vi "SMain.vi"() -> ()   [LabVIEW 2011] (continued)
-2.431327\t-2.435970\t-2.438255\t-2.439214\t-2.441636\t-2.442908\t-2.443591\t-2.444271\t-2.446042\t-2.447553\t-2.451574\t-2.454322\t-2.459259\t-2.459167\t-2.458988\t-2.459791\t-2.459803\t-2.460155\t-2.460693\t-2.460836\t-2.461752\t-2.464313\t-2.467197\t-2.467691\t-2.467576\t-2.466714\t-2.466182\t-2.465541\t-2.466343\t-2.466851\t-2.466728\t-2.468352\t-2.469074\t-2.468673\t-2.470402\t-2.472062\t-2.472489\t-2.471700\t-2.474044\t-2.476117\t-2.475176\t-2.475954\t-2.477194\t-2.478101\t-2.478769\t-2.482395\t-2.482993\t-2.485696\t-2.489882\t-2.491889\t-2.493382\t-2.496300\t-2.497217\t-2.495696\t-2.497921\t-2.498425\t-2.499485\t-2.502473\t-2.505013\t-2.507983\t-2.511344\t-2.514346\t-2.515093\t-2.515869\t-2.515267\t-2.517344\t-2.516297\t-2.517832\t-2.521177\t-2.524304\t-2.525843\t-2.529733\t-2.532366\t-2.533173\t-2.533271\t-2.533655\t-2.534038\t-2.534921\t-2.537768\t-2.538384\t-2.540839\t-2.543183\t-2.545565\t-2.547411\t-2.547801\t-2.550262\t-2.549876\t-2.551255\t-2.551288\t-2.551510\t-2.553730\t-2.556228\t-2.557870\t-2.560246\t-2.561557\t-2.564050\t-2.564885\t-2.566860\t-2.568948\t-2.568611\t-2.571201\t-2.573409\t-2.574788\t-2.577568\t-2.579327\t-2.581748\t-2.583365\t-2.586189\t-2.588238\t-2.588712\t-2.590200\t-2.592187\t-2.593757\t-2.594959\t-2.595729\t-2.597616\t-2.599509\t-2.602154\t-2.604658\t-2.607614\t-2.609660\t-2.610898\t-2.612830\t-2.613601\t-2.613473\t-2.613544\t-2.616515\t-2.620266\t-2.623817\t-2.625905\t-2.631148\t-2.636015\t-2.640186\t-2.641079\t-2.645126\t-2.645173\t-2.647065\t-2.649247\t-2.651238\t-2.654179\t-2.659284\t-2.665190\t-2.667742\t-2.672541\t-2.674807\t-2.673944\t-2.674205\t-2.673847\t-2.674862\t-2.676190\t-2.680985\t-2.685422\t-2.692200\t-2.698753\t-2.698318\t-2.697628\t-2.696863\t-2.697049\t-2.696832\t-2.697279\t-2.698751\t-2.702908\t-2.706973\t-2.710686\t-2.713145\t-2.713343\t-2.712896\t-2.711070\t-2.708909\t-2.707335\t-2.707843\t-2.708280\t-2.711253\t-2.715050\t-2.720516\t-2.723712\t-2.725368\t-2.726278\t-2.724675\t-2.723140\t-2.723831\t-2.722631\t-2.724579\t-2.727613\t-2.731521\t-2.734936\t-2.739656\t-2.743268\t-2.746792\t-2.750426\t-2.752496\t-2.755723\t-2.757728\t-2.759774\t-2.761461\t-2.765547\t-2.772756\t-2.778340\t-2.784959\t-2.791224\t-2.797387\t-2.800765\t-2.804883\t-2.808755\t-2.808718\t-2.813039\t-2.817153\t-2.823224\t-2.831411\t-2.838495\t-2.843969\t-2.849768\t-2.853002\t-2.856091\t-2.857814\t-2.858783\t-2.860619\t-2.865346\t-2.870363\t-2.877086\t-2.881230\t-2.886957\t-2.887244\t-2.886706\t-2.885127\t-2.880446\t-2.879572\t-2.879982\t-2.883966\t-2.885899\t-2.890801\t-2.894663\t-2.892103\t-2.888604\t-2.883640\t-2.878263\t-2.874808\t-2.869963\t-2.868088\t-2.865550\t-2.867525\t-2.869974\t-2.869190\t-2.870537\t-2.869512\t-2.866932\t-2.865189\t-2.861443"]
  in  "Impedance Spec String 2":string="@;@"
  in  "Data Points 2":i32
  in  "Compensation(ohm) 2":dbl
  in  "StopTimeNs 2":dbl
  in  "Start TimeNs 2":dbl
  in  "Impedance Filter 2":bool
  in  "Filter Risetime(ps) 2":dbl min=1.0 max=1000.0 step=1.0
  out "width2":i32
  out "width1":i32
  out "auto get refer point":bool
  out "SystemMode":string="GPF001"
  out "Count":i16=1
  out "DateCode8Value_0X30":i32=32 format="%x"
  out "ConvertStyle":bool
  out "CountXmlPath":path=path "D:/高频房软件/2. HPTS_VNA_Rev2.7.1.3-1107最新源码/DataBase/L99QF015-SD-R/20161114.xml"
  out "PassCount?":bool=TRUE
  out "upload":bool
  out "AlarmDisplay":bool=TRUE
  out "NetPathCompress2":path=path "\\\\172.20.20.113\\emc/HPTS/SI"
  out "NetPathCompress1":path=path "\\\\172.20.20.113\\emc/HPTS/VNA"
  out "NetCmdCompress":string="net use \\\\172.20.20.113 mesuser /user:mesuser"
  out "NetPathHW":string="\\\\172.20.20.86\\HuaweiData\\DataRoot\\XML"
  out "NetCmd":string="net use \\\\172.20.20.86 Luxshare-ict /user:C040345"
  out "NEXTList":string[](array[string])=["TX1-RX1", "TX2-RX1", "TX3-RX1", "TX4-RX1", "TX1-RX2", "TX2-RX2", "TX3-RX2", "TX4-RX2", "TX1-RX3", "TX2-RX3", "TX3-RX3", "TX4-RX3", "TX1-RX4", "TX2-RX4", "TX3-RX4", "TX4-RX4"]
  out "NEXTReults":bool[](array[boolean])
  out "SparaLists":string[](array[string])=["SDD21", "SDD11", "SCD22", "SCC11", "SCD21-SDD21", "ILD_15", "TDD11", "TDD22", "Pskew"]
  out "SparaReults":bool[](array[boolean])=[FALSE, FALSE, FALSE, FALSE, FALSE, TRUE, FALSE, FALSE, TRUE]
  out "FullXml":bool
  out "CustomerName":string="HuaWei"
  out "FileName":string="DevelopmentSystem"
  out "FileVersion":string="DevelopmentSystem"
  out "S写入延时（单位：ms） 2":dbl
  out "读取延时（单位：ms） 2":dbl
  out "Q写入延时（单位：ms） 2":dbl
  out "Test Status: 2":string="\n当前datacode为:0X20\n自动生成序列号小于本地MDB数据库记录SN，系统天数=数据库记录天数，生成流水号从数据库\n历史记录+1\nStart Test at 周一 上午 11:24:03 2016/11/14 China Time On wmg-PC.luxshare.com.cn\rP/N:L99QF015-SD-R,  Sample S/N:201611145014,  Length:1000mm\rThe Test Is Performed In Accordance With Related SI Spec\rS-parameter Testing.....\rSDD21_TX1:NG\rSDD11_TX1:NG\rSCD22_TX1:NG\rSCC11_TX1:NG\rSCD21-SDD21_TX1:NG\rTDD11_TX1:NG\rMax 133.38 117.59 \rMin 111.42 114.43 \rTDD22_TX1:NG\rMax 133.03 116.62 \rMin 109.85 113.82 \rTX1_Intra-pair Skew:0ps,OK (Spec max:15ps)\rSDD21_RX1:NG\rSDD11_RX1:NG\rSCD22_RX1:NG\rSCC11_RX1:NG\rSCD21-SDD21_RX1:NG\rTDD11_RX1:NG\rMax 128.10 116.52 \rMin 111.49 111.54 \rTDD22_RX1:NG\rMax 128.33 114.73 \rMin 108.98 109.00 \rRX1_Intra-pair Skew:0ps,OK (Spec max:15ps)\rSDD21_TX2:NG\rSDD11_TX2:NG\rSCD22_TX2:NG\rSCC11_TX2:NG\rSCD21-SDD21_TX2:NG\rTDD11_TX2:NG\rMax 129.55 115.75 \rMin 110.56 114.32 \rTDD22_TX2:NG\rMax 129.05 116.28 \rMin 108.99 114.50 \rTX2_Intra-pair Skew:0ps,OK (Spec max:15ps)\rSDD21_RX2:NG\rSDD11_RX2:NG\rSCD22_RX2:NG\rSCC11_RX2:NG\rSCD21-SDD21_RX2:NG\rTDD11_RX2:NG\rMax 129.31 117.05 \rMin 110.95 115.67 \rTDD22_RX2:NG\rMax 128.69 115.98 \rMin 110.50 114.65 \rRX2_Intra-pair Skew:0ps,OK (Spec max:15ps)\rSDD21_TX3:NG\rSDD11_TX3:NG\rSCD22_TX3:NG\rSCC11_TX3:NG\rSCD21-SDD21_TX3:NG\rTDD22_TX3:NG\rMax 133.03 114.43 \rMin 104.67 113.35 \rTDD11_TX3:NG\rMax 132.35 116.87 \rMin 104.39 115.18 \rTX3_Intra-pair Skew:0ps,OK (Spec max:15ps)\rSDD21_RX3:NG\rSDD11_RX3:NG\rSCD22_RX3:NG\rSCC11_RX3:NG\rSCD21-SDD21_RX3:NG\rTDD22_RX3:NG\rMax 127.53 115.30 \rMin 111.10 114.17 \rTDD11_RX3:NG\rMax 128.36 113.46 \rMin 109.35 111.72 \rRX3_Intra-pair Skew:0ps,OK (Spec max:15ps)\rSDD21_TX4:NG\rSDD11_TX4:NG\rSCD22_TX4:NG\rSCC11_TX4:NG\rSCD21-SDD21_TX4:NG\rTDD22_TX4:NG\rMax 128.13 114.91 \rMin 112.44 113.68 \rTDD11_TX4:NG\rMax 129.10 115.37 \rMin 111.66 113.97 \rTX4_Intra-pair Skew:0ps,OK (Spec max:15ps)\rSDD21_RX4:NG\rSDD11_RX4:NG\rSCD22_RX4:OK\rSCC11_RX4:NG\rSCD21-SDD21_RX4:NG\rTDD22_RX4:NG\rMax 133.06 117.74 \rMin 103.32 115.49 \rTDD11_RX4:NG\rMax 132.17 116.99 \rMin 102.07 114.63 \rRX4_Intra-pair Skew:0ps,OK (Spec max:15ps)\rSDD21_Total_Result:Fail\rSDD11_Total_Result:Fail\rSCD22_Total_Result:Fail\rSCC11_Total_Result:Fail\rSCD21-SDD21_Total_Result:Fail\rILD_15_Total_Result:Pass\rTDD11_Total_Result:Fail\rTDD22_Total_Result:Fail\rPskew_Total_Result:Pass\nWrite EEprom\nRead EEprom\nPort 0: FAIL\nPort 1: FAIL\nDemo mode Label has been printed!\n201611145014 :Test Finished !\rEnded Test At 周一 上午 11:25:36 2016/11/14 China Time.  Test Time: 93.165329s"
  out "未经进制转换的sn(客户 jin zhi sn)":string
  out "Shi jin zhi sn":string
  out "customer date":string
  out "S写入延时（单位：ms）":dbl=100.0
  out "读取延时（单位：ms）":dbl=100.0
  out "Q写入延时（单位：ms）":dbl=250.0
  out "要烧录的DateCode":string
  out "要烧录的时间和Sn":string
  out "strFSN 原始SN":string
  out "PRINT":refnum<k24>
  out "SN":refnum<k24>
  in  "labelConfig":string[](array[string])=["年周", "17", "18", "", "", "19", "20", "22", "22", "23", "27", "Z00A2Ryyww(X6)", "", "", "1", "0", ""]
  out "Go":bool
  out "cableType":string
  out "mid_str_descrip":string="年周"
  out "mid_array_temp_int":u8[][](array[numeric])=[[17, 6, 6, 0, 0, 0, 0, 0, 0, 0, 0, 0, 0, 0, 0, 0, 0, 0, 0, 0, 0, 0, 0, 0, 0, 0, 0, 0, 0, 0, 0, 0, 0, 0, 0, 0, 0, 0, 0, 0, 0, 0, 0, 0, 0, 0, 0, 0, 0, 0, 0, 0, 0, 0, 0, 0, 0, 0, 0, 0, 0, 0, 0, 0, 0, 0, 0, 0, 0, 0, 0, 0, 0, 0, 0, 0, 0, 0, 0, 0, 0, 0, 0, 0, 0, 0, 0, 0, 0, 0, 0, 0, 0, 0, 0, 0, 0, 0, 0, 0, 0, 0, 0, 0, 0, 0, 0, 0, 0, 0, 56, 0, 0, 0, 0, 0, 0, 0, 0, 0, 0, 0, 0, 0, 0, 0, 0, 0, 17, 0, 35, 136, 0, 0, 0, 0, 0, 128, 0, 5, 255, 0, 0, 0, 0, 0, 1, 160, 76, 85, 88, 83, 72, 65, 82, 69, 45, 73, 67, 84, 32, 32, 32, 32, 31, 60, 24, 160, 76, 57, 57, 81, 70, 48, 49, 53, 45, 83, 68, 45, 82, 32, 32, 32, 66, 32, 3, 4, 5, 8, 70, 55, 11, 0, 0, 0, 90, 48, 48, 65, 50, 82, 49, 54, 52, 55, 48, 48, 53, 48, 49, 56, 49, 54, 49, 49, 49, 52, 32, 32, 0, 0, 103, 95, 0, 0, 0, 0, 0, 0, 0, 0, 0, 0, 0, 0, 0, 0, 0, 0, 0, 0, 0, 0, 0, 0, 0, 0, 0, 0, 0, 0, 0, 0, 0, 0], [17, 6, 6, 0, 0, 0, 0, 0, 0, 0, 0, 0, 0, 0, 0, 0, 0, 0, 0, 0, 0, 0, 0, 0, 0, 0, 0, 0, 0, 0, 0, 0, 0, 0, 0, 0, 0, 0, 0, 0, 0, 0, 0, 0, 0, 0, 0, 0, 0, 0, 0, 0, 0, 0, 0, 0, 0, 0, 0, 0, 0, 0, 0, 0, 0, 0, 0, 0, 0, 0, 0, 0, 0, 0, 0, 0, 0, 0, 0, 0, 0, 0, 0, 0, 0, 0, 0, 0, 0, 0, 0, 0, 0, 0, 0, 0, 0, 0, 0, 0, 0, 0, 0, 0, 0, 0, 0, 0, 0, 0, 56, 0, 0, 0, 0, 0, 0, 0, 0, 0, 0, 0, 0, 0, 0, 0, 0, 0, 17, 0, 35, 136, 0, 0, 0, 0, 0, 128, 0, 5, 255, 0, 0, 0, 0, 0, 1, 160, 76, 85, 88, 83, 72, 65, 82, 69, 45, 73, 67, 84, 32, 32, 32, 32, 31, 60, 24, 160, 76, 57, 57, 81, 70, 48, 49, 53, 45, 83, 68, 45, 82, 32, 32, 32, 66, 32, 3, 4, 5, 8, 70, 55, 11, 0, 0, 0, 90, 48, 48, 65, 50, 82, 49, 54, 52, 55, 48, 48, 53, 48, 49, 56, 49, 54, 49, 49, 49, 52, 32, 32, 0, 0, 103, 95, 0, 0, 0, 0, 0, 0, 0, 0, 0, 0, 0, 0, 0, 0, 0, 0, 0, 0, 0, 0, 0, 0, 0, 0, 0, 0, 0, 0, 0, 0, 0, 0]] format="%.0x"
  out "mid_str_snformat":string="Z00A2Ryyww(X6)"
  out "mid_str_labelType":string="QSFP+28_HW"
  out "mid_array_eep":string[][](array[string])=[["11", "11"], ["6", "6"], ["6", "6"], ["0", "0"], ["0", "0"], ["0", "0"], ["0", "0"], ["0", "0"], ["0", "0"], ["0", "0"], ["0", "0"], ["0", "0"], ["0", "0"], ["0", "0"], ["0", "0"], ["0", "0"], ["0", "0"], ["0", "0"], ["0", "0"], ["0", "0"], ["0", "0"], ["0", "0"], ["0", "0"], ["0", "0"], ["0", "0"], ["0", "0"], ["0", "0"], ["0", "0"], ["0", "0"], ["0", "0"], ["0", "0"], ["0", "0"], ["0", "0"], ["0", "0"], ["0", "0"], ["0", "0"], ["0", "0"], ["0", "0"], ["0", "0"], ["0", "0"], ["0", "0"], ["0", "0"], ["0", "0"], ["0", "0"], ["0", "0"], ["0", "0"], ["0", "0"], ["0", "0"], ["0", "0"], ["0", "0"], ["0", "0"], ["0", "0"], ["0", "0"], ["0", "0"], ["0", "0"], ["0", "0"], ["0", "0"], ["0", "0"], ["0", "0"], ["0", "0"], ["0", "0"], ["0", "0"], ["0", "0"], ["0", "0"], ["0", "0"], ["0", "0"], ["0", "0"], ["0", "0"], ["0", "0"], ["0", "0"], ["0", "0"], ["0", "0"], ["0", "0"], ["0", "0"], ["0", "0"], ["0", "0"], ["0", "0"], ["0", "0"], ["0", "0"], ["0", "0"], ["0", "0"], ["0", "0"], ["0", "0"], ["0", "0"], ["0", "0"], ["0", "0"], ["0", "0"], ["0", "0"], ["0", "0"], ["0", "0"], ["0", "0"], ["0", "0"], ["0", "0"], ["0", "0"], ["0", "0"], ["0", "0"], ["0", "0"], ["0", "0"], ["0", "0"], ["0", "0"], ["0", "0"], ["0", "0"], ["0", "0"], ["0", "0"], ["0", "0"], ["0", "0"], ["0", "0"], ["0", "0"], ["0", "0"], ["0", "0"], ["38", "38"], ["0", "0"], ["0", "0"], ["0", "0"], ["0", "0"], ["0", "0"], ["0", "0"], ["0", "0"], ["0", "0"], ["0", "0"], ["0", "0"], ["0", "0"], ["0", "0"], ["0", "0"], ["0", "0"], ["0", "0"], ["0", "0"], ["0", "0"], ["11", "11"], ["0", "0"], ["23", "23"], ["88", "88"], ["0", "0"], ["0", "0"], ["0", "0"], ["0", "0"], ["0", "0"], ["80", "80"], ["0", "0"], ["5", "5"], ["FF", "FF"], ["0", "0"], ["0", "0"], ["0", "0"], ["0", "0"], ["0", "0"], ["1", "1"], ["A0", "A0"], ["4C", "4C"], ["55", "55"], ["58", "58"], ["53", "53"], ["48", "48"], ["41", "41"], ["52", "52"], ["45", "45"], ["2D", "2D"], ["49", "49"], ["43", "43"], ["54", "54"], ["20", "20"], ["20", "20"], ["20", "20"], ["20", "20"], ["1F", "1F"], ["3C", "3C"], ["18", "18"], ["A0", "A0"], ["4C", "4C"], ["39", "39"], ["39", "39"], ["51", "51"], ["46", "46"], ["30", "30"], ["31", "31"], ["35", "35"], ["2D", "2D"], ["53", "53"], ["44", "44"], ["2D", "2D"], ["52", "52"], ["20", "20"], ["20", "20"], ["20", "20"], ["42", "42"], ["20", "20"], ["3", "3"], ["4", "4"], ["5", "5"], ["8", "8"], ["46", "46"], ["0", "0"], ["0B", "0B"], ["0", "0"], ["0", "0"], ["0", "0"], ["5A", "5A"], ["30", "30"], ["30", "30"], ["41", "41"], ["32", "32"], ["52", "52"], ["20", "20"], ["20", "20"], ["20", "20"], ["20", "20"], ["20", "20"], ["20", "20"], ["20", "20"], ["20", "20"], ["20", "20"], ["20", "20"], ["20", "20"], ["20", "20"], ["20", "20"], ["20", "20"], ["20", "20"], ["20", "20"], ["20", "20"], ["20", "20"], ["0", "0"], ["0", "0"], ["67", "67"], ["0", "0"], ["0", "0"], ["0", "0"], ["0", "0"], ["0", "0"], ["0", "0"], ["0", "0"], ["0", "0"], ["0", "0"], ["0", "0"], ["0", "0"], ["0", "0"], ["0", "0"], ["0", "0"], ["0", "0"], ["0", "0"], ["0", "0"], ["0", "0"], ["0", "0"], ["0", "0"], ["0", "0"], ["0", "0"], ["0", "0"], ["0", "0"], ["0", "0"], ["0", "0"], ["0", "0"], ["0", "0"], ["0", "0"], ["0", "0"], ["0", "0"], ["0", "0"], ["0", "0"]]
  out "测试项目及频点在txt输出":string="$\nSDD21 TX1\n           RX1\n           TX2\n           RX2\n           TX3\n           RX3\n           TX4\n           RX4 #\nSDD11 TX1\n           RX1\n           TX2\n           RX2\n           TX3\n           RX3\n           TX4\n           RX4 #\nSCD22 TX1\n           RX1\n           TX2\n           RX2\n           TX3\n           RX3\n           TX4\n           RX4 #\nSCC11 TX1\n           RX1\n           TX2\n           RX2\n           TX3\n           RX3\n           TX4\n           RX4 #\nSCD21-SDD21 TX1\n           RX1\n           TX2\n           RX2\n           TX3\n           RX3\n           TX4\n           RX4 #\nILD_15 TX1\n           RX1\n           TX2\n           RX2\n           TX3\n           RX3\n           TX4\n           RX4 #$\n"
  out "txt summary":string="\n当前datacode为:0X20\n自动生成序列号小于本地MDB数据库记录SN，系统天数=数据库记录天数，生成流水号从数据库\n历史记录+1\nStart Test at 周一 上午 11:24:03 2016/11/14 China Time On wmg-PC.luxshare.com.cn\rP/N:L99QF015-SD-R,  Sample S/N:201611145014,  Length:1000mm\rThe Test Is Performed In Accordance With Related SI Spec\rS-parameter Testing.....\rSDD21_TX1:NG\rSDD11_TX1:NG\rSCD22_TX1:NG\rSCC11_TX1:NG\rSCD21-SDD21_TX1:NG\rTDD11_TX1:NG\rMax 133.38 117.59 \rMin 111.42 114.43 \rTDD22_TX1:NG\rMax 133.03 116.62 \rMin 109.85 113.82 \rTX1_Intra-pair Skew:0ps,OK (Spec max:15ps)\rSDD21_RX1:NG\rSDD11_RX1:NG\rSCD22_RX1:NG\rSCC11_RX1:NG\rSCD21-SDD21_RX1:NG\rTDD11_RX1:NG\rMax 128.10 116.52 \rMin 111.49 111.54 \rTDD22_RX1:NG\rMax 128.33 114.73 \rMin 108.98 109.00 \rRX1_Intra-pair Skew:0ps,OK (Spec max:15ps)\rSDD21_TX2:NG\rSDD11_TX2:NG\rSCD22_TX2:NG\rSCC11_TX2:NG\rSCD21-SDD21_TX2:NG\rTDD11_TX2:NG\rMax 129.55 115.75 \rMin 110.56 114.32 \rTDD22_TX2:NG\rMax 129.05 116.28 \rMin 108.99 114.50 \rTX2_Intra-pair Skew:0ps,OK (Spec max:15ps)\rSDD21_RX2:NG\rSDD11_RX2:NG\rSCD22_RX2:NG\rSCC11_RX2:NG\rSCD21-SDD21_RX2:NG\rTDD11_RX2:NG\rMax 129.31 117.05 \rMin 110.95 115.67 \rTDD22_RX2:NG\rMax 128.69 115.98 \rMin 110.50 114.65 \rRX2_Intra-pair Skew:0ps,OK (Spec max:15ps)\rSDD21_TX3:NG\rSDD11_TX3:NG\rSCD22_TX3:NG\rSCC11_TX3:NG\rSCD21-SDD21_TX3:NG\rTDD22_TX3:NG\rMax 133.03 114.43 \rMin 104.67 113.35 \rTDD11_TX3:NG\rMax 132.35 116.87 \rMin 104.39 115.18 \rTX3_Intra-pair Skew:0ps,OK (Spec max:15ps)\rSDD21_RX3:NG\rSDD11_RX3:NG\rSCD22_RX3:NG\rSCC11_RX3:NG\rSCD21-SDD21_RX3:NG\rTDD22_RX3:NG\rMax 127.53 115.30 \rMin 111.10 114.17 \rTDD11_RX3:NG\rMax 128.36 113.46 \rMin 109.35 111.72 \rRX3_Intra-pair Skew:0ps,OK (Spec max:15ps)\rSDD21_TX4:NG\rSDD11_TX4:NG\rSCD22_TX4:NG\rSCC11_TX4:NG\rSCD21-SDD21_TX4:NG\rTDD22_TX4:NG\rMax 128.13 114.91 \rMin 112.44 113.68 \rTDD11_TX4:NG\rMax 129.10 115.37 \rMin 111.66 113.97 \rTX4_Intra-pair Skew:0ps,OK (Spec max:15ps)\rSDD21_RX4:NG\rSDD11_RX4:NG\rSCD22_RX4:OK\rSCC11_RX4:NG\rSCD21-SDD21_RX4:NG\rTDD22_RX4:NG\rMax 133.06 117.74 \rMin 103.32 115.49 \rTDD11_RX4:NG\rMax 132.17 116.99 \rMin 102.07 114.63 \rRX4_Intra-pair Skew:0ps,OK (Spec max:15ps)\rSDD21_Total_Result:Fail\rSDD11_Total_Result:Fail\rSCD22_Total_Result:Fail\rSCC11_Total_Result:Fail\rSCD21-SDD21_Total_Result:Fail\rILD_15_Total_Result:Pass\rTDD11_Total_Result:Fail\rTDD22_Total_Result:Fail\rPskew_Total_Result:Pass\nWrite EEprom\nRead EEprom\nPort 0: FAIL\nPort 1: FAIL\nDemo mode Label has been printed!\n201611145014 :Test Finished !$\nSDD21 TX1\n           RX1\n           TX2\n           RX2\n           TX3\n           RX3\n           TX4\n           RX4 #\nSDD11 TX1\n           RX1\n           TX2\n           RX2\n           TX3\n           RX3\n           TX4\n           RX4 #\nSCD22 TX1\n           RX1\n           TX2\n           RX2\n           TX3\n           RX3\n           TX4\n           RX4 #\nSCC11 TX1\n           RX1\n           TX2\n           RX2\n           TX3\n           RX3\n           TX4\n           RX4 #\nSCD21-SDD21 TX1\n           RX1\n           TX2\n           RX2\n           TX3\n           RX3\n           TX4\n           RX4 #\nILD_15 TX1\n           RX1\n           TX2\n           RX2\n           TX3\n           RX3\n           TX4\n           RX4 #$\n\rEnded Test At 周一 上午 11:25:36 2016/11/14 China Time.  Test Time: 93.165329s\nswitch status:demo or manual mode"
  out "frePoints":string[](array[string])
  in  "nCmdShow":i16(ring) items=["SW_HIDE   ", "SW_SHOWNORMAL", "SW_SHOWMINIMIZED", "SW_SHOWMAXIMIZED", "SW_SHOWNOACTIVATE", "SW_SHOW", "SW_MINIMIZE", "SW_SHOWMINNOACTIVE", "SW_SHOWNA", "SW_RESTORE"]
  out "proBar_ref":refnum<vi>
  out "AutoSN":bool=TRUE
  out "show_impspec":string[](array[string])
  out "show_Next":string[](array[string])
  out "show_TDD22":string[](array[string])
  out "show_ILD":string[](array[string])
  out "show_SCC11":string[](array[string])
  out "show_SDD11":string[](array[string])
  out "show_SDD21":string[](array[string])
  out "show_TDD11":string[](array[string])
  out "labelFlag":bool
  out "Cus":string="HuaWei"
  in  "imp_cable spec":string
  in  "imp_term spec":string
  in  "test time":string[](array[string])=["2016/11/14 11:59:03"]
  out "show_date_test":timestamp=timestamp(3527207877 s since 1904-01-01) format="%<%x>T"
  out "midVar_str_SN":string="5018"
  out "midVar_time_date":timestamp=timestamp(3561940740.543268 s since 1904-01-01)
  in  "midVar_bool_find":bool=TRUE
  out "EEResult":bool
  out "条码输出":string
  in  "State":string="wait"
  out "upload":bool
  in  "read port0":string[][](array[string])
  in  "read port2":string[][](array[string])
  in  "read port3":string[][](array[string])
  in  "read port4":string[][](array[string])
  in  "read port1":string[][](array[string])
  out "ref_read_ports":refnum<vi>[](array[refnum])
  out "ref_temp_ports":refnum<vi>[](array[refnum])
  in  "temp port1":string[][](array[string])
  in  "temp port4":string[][](array[string])
  in  "temp port3":string[][](array[string])
  in  "temp port2":string[][](array[string])
  in  "temp port0":string[][](array[string])
  out "Label Type":string[](array[string])
  out "Data In":string[](array[string])=["L99QF015-SD-R", "30", "", "", ""]
  out "LabelTF":bool=TRUE
  out "EEPROMTF":bool=TRUE
  out "start":timestamp=timestamp(3561940743.152417 s since 1904-01-01)
  out "db_SI":string
  out "db_VNA":string="L99QF015-SD-R;201611145018;"
  in  "db_ResultString":string="SDD21_TX1:NG,SDD11_TX1:NG,SCD22_TX1:NG,SCC11_TX1:NG,SCD21-SDD21_TX1:NG,TDD11_TX1:NG,Max 133.38 117.59 ,Min 111.42 114.43 ,TDD22_TX1:NG,Max 133.03 116.62 ,Min 109.85 113.82 ,TX1_Intra-pair Skew:0ps,OK (Spec max:15ps),SDD21_RX1:NG,SDD11_RX1:NG,SCD22_RX1:NG,SCC11_RX1:NG,SCD21-SDD21_RX1:NG,TDD11_RX1:NG,Max 128.10 116.52 ,Min 111.49 111.54 ,TDD22_RX1:NG,Max 128.33 114.73 ,Min 108.98 109.00 ,RX1_Intra-pair Skew:0ps,OK (Spec max:15ps),SDD21_TX2:NG,SDD11_TX2:NG,SCD22_TX2:NG,SCC11_TX2:NG,SCD21-SDD21_TX2:NG,TDD11_TX2:NG,Max 129.55 115.75 ,Min 110.56 114.32 ,TDD22_TX2:NG,Max 129.05 116.28 ,Min 108.99 114.50 ,TX2_Intra-pair Skew:0ps,OK (Spec max:15ps),SDD21_RX2:NG,SDD11_RX2:NG,SCD22_RX2:NG,SCC11_RX2:NG,SCD21-SDD21_RX2:NG,TDD11_RX2:NG,Max 129.31 117.05 ,Min 110.95 115.67 ,TDD22_RX2:NG,Max 128.69 115.98 ,Min 110.50 114.65 ,RX2_Intra-pair Skew:0ps,OK (Spec max:15ps),SDD21_TX3:NG,SDD11_TX3:NG,SCD22_TX3:NG,SCC11_TX3:NG,SCD21-SDD21_TX3:NG,TDD22_TX3:NG,Max 133.03 114.43 ,Min 104.67 113.35 ,TDD11_TX3:NG,Max 132.35 116.87 ,Min 104.39 115.18 ,TX3_Intra-pair Skew:0ps,OK (Spec max:15ps),SDD21_RX3:NG,SDD11_RX3:NG,SCD22_RX3:NG,SCC11_RX3:NG,SCD21-SDD21_RX3:NG,TDD22_RX3:NG,Max 127.53 115.30 ,Min 111.10 114.17 ,TDD11_RX3:NG,Max 128.36 113.46 ,Min 109.35 111.72 ,RX3_Intra-pair Skew:0ps,OK (Spec max:15ps),SDD21_TX4:NG,SDD11_TX4:NG,SCD22_TX4:NG,SCC11_TX4:NG,SCD21-SDD21_TX4:NG,TDD22_TX4:NG,Max 128.13 114.91 ,Min 112.44 113.68 ,TDD11_TX4:NG,Max 129.10 115.37 ,Min 111.66 113.97 ,TX4_Intra-pair Skew:0ps,OK (Spec max:15ps),SDD21_RX4:NG,SDD11_RX4:NG,SCD22_RX4:OK,SCC11_RX4:NG,SCD21-SDD21_RX4:NG,TDD22_RX4:NG,Max 133.06 117.74 ,Min 103.32 115.49 ,TDD11_RX4:NG,Max 132.17 116.99 ,Min 102.07 114.63 ,RX4_Intra-pair Skew:0ps,OK (Spec max:15ps),NEXT_TX1-RX1:NG,NEXT_TX2-RX1:NG,NEXT_TX3-RX1:NG,NEXT_TX4-RX1:NG,NEXT_TX1-RX2:NG,NEXT_TX2-RX2:NG,NEXT_TX3-RX2:NG,NEXT_TX4-RX2:NG,NEXT_TX1-RX3:NG,NEXT_TX2-RX3:NG,NEXT_TX3-RX3:NG,NEXT_TX4-RX3:NG,NEXT_TX1-RX4:NG,NEXT_TX2-RX4:NG,NEXT_TX3-RX4:NG,NEXT_TX4-RX4:NG,$SDD21_TX1:SDD21_RX1:SDD21_TX2:SDD21_RX2:SDD21_TX3:SDD21_RX3:SDD21_TX4:SDD21_RX4 #:SDD11_TX1:SDD11_RX1:SDD11_TX2:SDD11_RX2:SDD11_TX3:SDD11_RX3:SDD11_TX4:SDD11_RX4 #:SCD22_TX1:SCD22_RX1:SCD22_TX2:SCD22_RX2:SCD22_TX3:SCD22_RX3:SCD22_TX4:SCD22_RX4 #:SCC11_TX1:SCC11_RX1:SCC11_TX2:SCC11_RX2:SCC11_TX3:SCC11_RX3:SCC11_TX4:SCC11_RX4 #:SCD21-SDD21_TX1:SCD21-SDD21_RX1:SCD21-SDD21_TX2:SCD21-SDD21_RX2:SCD21-SDD21_TX3:SCD21-SDD21_RX3:SCD21-SDD21_TX4:SCD21-SDD21_RX4 #:ILD_15_TX1:ILD_15_RX1:ILD_15_TX2:ILD_15_RX2:ILD_15_TX3:ILD_15_RX3:ILD_15_TX4:ILD_15_RX4 #$"
  out "Option":T11={"Urgent Stop"=FALSE, "Crosstalk  by Trace"=FALSE, "Dem 2X"=TRUE, "2X equalize "=FALSE}
  out "TDR Setting":T12={"Start TimeNs"=0.0, "StopTimeNs"=5.0, "Data Points"=4000, "Compensation(ohm)"=0.0, "DataFormat"=6, "Impedance Filter"=TRUE, "Filter Risetime(ps)"=30.0, "Impedance Spec String"="0.75@110@2@110;0.75@90@2@95", "Skew Spec(ps)"=15, "CMP setting"=""}
  out "Skew Spec(ps)":i32=15
  out "2X IL":dbl[](array[numeric])=[-0.025299, -0.038396, -0.047424, -0.055976, -0.059331, -0.068781, -0.07578, -0.081239, -0.089022, -0.093241, -0.097614, -0.102462, -0.106838, -0.111812, -0.116556, -0.121163, -0.12561, -0.131718, -0.134792, -0.13877, -0.145469, -0.149479, -0.152659, -0.157142, -0.162291, -0.164771, -0.168818, -0.17033, -0.176722, -0.179419, -0.183921, -0.186601, -0.190951, -0.193378, -0.19824, -0.20176, -0.202689, -0.207947, -0.211354, -0.214498, -0.220736, -0.223214, -0.225991, -0.227897, -0.231621, -0.235236, -0.238474, -0.242007, -0.244427, -0.24856, -0.251615, -0.255644, -0.257638, -0.261234, -0.264621, -0.266303, -0.269738, -0.272241, -0.274441, -0.276158, -0.279938, -0.282564, -0.28537, -0.288029, -0.292169, -0.294557, -0.297687, -0.301761, -0.304652, -0.305833, -0.307066, -0.309591, -0.312562, -0.315843, -0.31639, -0.31604, -0.318513, -0.320032, -0.322668, -0.32612, -0.330335, -0.334297, -0.34034, -0.341411, -0.345104, -0.347321, -0.349213, -0.351984, -0.354782, -0.356899, -0.357019, -0.361617, -0.362734, -0.36572, -0.367166, -0.371019, -0.372807, -0.37617, -0.378489, -0.380671, -0.383681, -0.385224, -0.386151, -0.388422, -0.389343, -0.39172, -0.393825, -0.397043, -0.398343, -0.400077, -0.405011, -0.406109, -0.409167, -0.410383, -0.411453, -0.41508, -0.417531, -0.419854, -0.421583, -0.424947, -0.42654, -0.429572, -0.430897, -0.434433, -0.435632, -0.438249, -0.440184, -0.442646, -0.444562, -0.445842, -0.447651, -0.450634, -0.452453, -0.454341, -0.457792, -0.459201, -0.460308, -0.461669, -0.462777, -0.464409, -0.468144, -0.470502, -0.47275, -0.475034, -0.475669, -0.478023, -0.478382, -0.480829, -0.482842, -0.484459, -0.486674, -0.489177, -0.491121, -0.494005, -0.495936, -0.497061, -0.499267, -0.50051, -0.502804, -0.50405, -0.505765, -0.507052, -0.509473, -0.512389, -0.51437, -0.515671, -0.517533, -0.519425, -0.52189, -0.521842, -0.52303, -0.525679, -0.528968, -0.530579, -0.532575, -0.53465, -0.536459, -0.537934, -0.539202, -0.54086, -0.542603, -0.5457, -0.547524, -0.548774, -0.549721, -0.552302, -0.554863, -0.556646, -0.559567, -0.560755, -0.564216, -0.565447, -0.56634, -0.567621, -0.568795, -0.572849, -0.573837, -0.573788, -0.575949, -0.580124, -0.580805, -0.583633, -0.584421, -0.586743, -0.588333, -0.590903, -0.592009, -0.594853, -0.595409, -0.597326, -0.596798, -0.597763, -0.60116, -0.60416, -0.606395, -0.609768, -0.610518, -0.612809, -0.614324, -0.616136, -0.617459, -0.618913, -0.618354, -0.620853, -0.624932, -0.626581, -0.630236, -0.632642, -0.633388, -0.63542, -0.635927, -0.636904, -0.638461, -0.640481, -0.642285, -0.643035, -0.645007, -0.647452, -0.650336, -0.650522, -0.650374, -0.652932, -0.654354, -0.6563, -0.657573, -0.660404, -0.661557, -0.664981, -0.665852, -0.666908, -0.670274, -0.671692, -0.672849, -0.675964, -0.679116, -0.680009, -0.680817, -0.682485, -0.684064, -0.685281, -0.685714, -0.689176, -0.689231, -0.691987, -0.693946, -0.696069, -0.697712, -0.700794, -0.701734, -0.703201, -0.703776, -0.705657, -0.708378, -0.71062, -0.711792, -0.713659, -0.715097, -0.716667, -0.718491, -0.720789, -0.721948, -0.722241, -0.724976, -0.726849, -0.72666, -0.729363, -0.730162, -0.732883, -0.735904, -0.736952, -0.739038, -0.73981, -0.741586, -0.743353, -0.745631, -0.747878, -0.748821, -0.750045, -0.751315, -0.75408, -0.756592, -0.758178, -0.759658, -0.76182, -0.762632, -0.764898, -0.765885, -0.768208, -0.769777, -0.771565, -0.77349, -0.77466, -0.77747, -0.77947, -0.780437, -0.783258, -0.784929, -0.787219, -0.78773, -0.789671, -0.791426, -0.793443, -0.795477, -0.798215, -0.798336, -0.800847, -0.801219, -0.804592, -0.804967, -0.807604, -0.808648, -0.811207, -0.812119, -0.814463, -0.816479, -0.816857, -0.818916, -0.820631, -0.82228, -0.824061, -0.826539, -0.829216, -0.830524, -0.832218, -0.833493, -0.834462, -0.836032, -0.838399, -0.839965, -0.843226, -0.842684, -0.844971, -0.848181, -0.849788, -0.85147, -0.853466, -0.8544, -0.856009, -0.85821, -0.860153, -0.862614, -0.863089, -0.865995, -0.866916, -0.869606, -0.87226, -0.872654, -0.873102, -0.874217, -0.875987, -0.878471, -0.880127, -0.881265, -0.883254, -0.885726, -0.887636, -0.888446, -0.889525, -0.89144, -0.89356, -0.895586, -0.89772, -0.898394, -0.901539, -0.902978, -0.903626, -0.905436, -0.907707, -0.908756, -0.91031, -0.911702, -0.913224, -0.914065, -0.915603, -0.917613, -0.918547, -0.920796, -0.921613, -0.925115, -0.926152, -0.927588, -0.930169, -0.931709, -0.932481, -0.934098, -0.936424, -0.936876, -0.937659, -0.939378, -0.941622, -0.943235, -0.942614, -0.945728, -0.946817, -0.949055, -0.95112, -0.95217, -0.955136, -0.957149, -0.957272, -0.959033, -0.9612, -0.961962, -0.963545, -0.967061, -0.968399, -0.970546, -0.973385, -0.973856, -0.974207, -0.975643, -0.97884, -0.97915, -0.980188, -0.982034, -0.98472, -0.986456, -0.988529, -0.989871, -0.992863, -0.994155, -0.996464, -0.998286, -0.999287, -1.000963, -1.001043, -1.002651, -1.00456, -1.007629, -1.008066, -1.009819, -1.01113, -1.013663, -1.014789, -1.017072, -1.019742, -1.021611, -1.023713, -1.025332, -1.026222, -1.026869, -1.027743, -1.030052, -1.03073, -1.033045, -1.035049, -1.036088, -1.03854, -1.041763, -1.042051, -1.043345, -1.044835, -1.045911, -1.047474, -1.050112, -1.050947, -1.054054, -1.056098, -1.056999, -1.058949, -1.060286, -1.061237, -1.061735, -1.064154, -1.066454, -1.068678, -1.068777, -1.071732, -1.07341, -1.073918, -1.07718, -1.078266, -1.080347, -1.081876, -1.083674, -1.084348, -1.085916, -1.086228, -1.089243, -1.090434, -1.091868, -1.094835, -1.096616, -1.096945, -1.099785, -1.102174, -1.103444, -1.10423, -1.105284, -1.106884, -1.107956, -1.108242, -1.110338, -1.113661, -1.114571, -1.117028, -1.118751, -1.119113, -1.121022, -1.123104, -1.122807, -1.125616, -1.127797, -1.12873, -1.12972, -1.132328, -1.133934, -1.136053, -1.13791, -1.138532, -1.139899, -1.141078, -1.142651, -1.141653, -1.145035, -1.146205, -1.147698, -1.149198, -1.151227, -1.15306, -1.155051, -1.157576, -1.158307, -1.160585, -1.161081, -1.162078, -1.164421, -1.165552, -1.167357, -1.16903, -1.16941, -1.172091, -1.173558, -1.175417, -1.177655, -1.179563, -1.180398, -1.181254, -1.183122, -1.184561, -1.185409, -1.186553, -1.188506, -1.190284, -1.19296, -1.194518, -1.196114, -1.199446, -1.199928, -1.201659, -1.203025, -1.204984, -1.205929, -1.207424, -1.20884, -1.212338, -1.213546, -1.216908, -1.219662, -1.222377, -1.223413, -1.224234, -1.224444, -1.226533, -1.227726, -1.229907, -1.230216, -1.233822, -1.235221, -1.23743, -1.238272, -1.239472, -1.240008, -1.241383, -1.242313, -1.244294, -1.245158, -1.247334, -1.248006, -1.250743, -1.251832, -1.252133, -1.253227, -1.255278, -1.256617, -1.257998, -1.258347, -1.259462, -1.262189, -1.26538, -1.265117, -1.267315, -1.267774, -1.269888, -1.271996, -1.272938, -1.272988, -1.276344, -1.278889, -1.280114, -1.282203, -1.282807, -1.2851, -1.286312, -1.28754, -1.289422, -1.290962, -1.293184, -1.295772, -1.297139, -1.300557, -1.30177, -1.303345, -1.303985, -1.306281, -1.307709, -1.309835, -1.309741, -1.312592, -1.315234, -1.317538, -1.319714, -1.322086, -1.323841, -1.32463, -1.326073, -1.327763, -1.329139, -1.329624, -1.331755, -1.332977, -1.33489, -1.33754, -1.339253, -1.342017, -1.344422, -1.345122, -1.345541, -1.346031, -1.346359, -1.3474, -1.348735, -1.349061, -1.350116, -1.353398, -1.354305, -1.357842, -1.356693, -1.358147, -1.359578, -1.360392, -1.361354, -1.363513, -1.364167, -1.365032, -1.366879, -1.367457, -1.368583, -1.370459, -1.371694, -1.373734, -1.376242, -1.379085, -1.379925, -1.379883, -1.381184, -1.381655, -1.38242, -1.38571, -1.387976, -1.390893, -1.394178, -1.396827, -1.399715, -1.402093, -1.404467, -1.404706, -1.405469, -1.407391, -1.409543, -1.41276, -1.414513, -1.419863, -1.421498, -1.423363, -1.425305, -1.426751, -1.426783, -1.428077, -1.428979, -1.43197, -1.434989, -1.437283, -1.438178, -1.440308, -1.441654, -1.442987, -1.443577, -1.44396, -1.443438, -1.445594, -1.44515, -1.445881, -1.448352, -1.449836, -1.450411, -1.451182, -1.452277, -1.453172, -1.453119, -1.453, -1.453989, -1.456489, -1.456532, -1.458466, -1.458938, -1.460769, -1.462027, -1.462978, -1.462454, -1.464558, -1.46441, -1.466658, -1.466867, -1.468869, -1.47093, -1.472731, -1.47355, -1.474344, -1.474451, -1.476897, -1.478554, -1.479486, -1.481271, -1.483897, -1.484711, -1.487268, -1.488311, -1.489221, -1.49104, -1.491298, -1.491559, -1.493292, -1.496642, -1.497452, -1.499759, -1.501398, -1.502206, -1.506306, -1.506314, -1.508587, -1.509562, -1.51105, -1.511548, -1.514521, -1.516246, -1.518962, -1.522518, -1.52399, -1.526348, -1.526897, -1.529924, -1.531145, -1.532163, -1.533655, -1.534977, -1.536481, -1.538672, -1.541062, -1.542947, -1.544094, -1.543103, -1.545053, -1.546173, -1.547124, -1.548823, -1.550699, -1.552797, -1.552814, -1.553599, -1.555463, -1.557036, -1.556812, -1.559025, -1.557934, -1.559971, -1.563383, -1.565346, -1.567625, -1.568344, -1.569628, -1.571566, -1.571053, -1.572094, -1.571631, -1.575197, -1.576725, -1.579283, -1.580539, -1.582093, -1.583907, -1.58632, -1.587807, -1.589771, -1.590995, -1.591517, -1.593725, -1.595636, -1.596745, -1.596782, -1.598313, -1.601373, -1.600936, -1.602629, -1.605288, -1.606105, -1.608735, -1.609487, -1.612002, -1.612291, -1.612418, -1.615246, -1.612903, -1.614471, -1.615906, -1.618467, -1.619485, -1.621517, -1.623681, -1.626157, -1.6257, -1.627696, -1.629418, -1.631466, -1.632745, -1.633825, -1.636445, -1.639073, -1.640156, -1.642296, -1.642965, -1.644254, -1.646067, -1.645605, -1.647812, -1.648925, -1.650588, -1.653483, -1.654076, -1.655474, -1.656504, -1.659452, -1.660971, -1.661502, -1.661876, -1.66426, -1.665877, -1.665611, -1.668485, -1.66745, -1.668267, -1.668875, -1.670443, -1.671893, -1.673731, -1.676482, -1.677827, -1.679732, -1.68129, -1.681868, -1.684248, -1.687335, -1.689643, -1.691646, -1.693701, -1.696813, -1.699129, -1.699837, -1.700024, -1.702098, -1.704938, -1.708093, -1.709145, -1.712602, -1.715345, -1.717833, -1.720597, -1.721398, -1.723556, -1.72594, -1.726716, -1.726466, -1.72838, -1.729853, -1.729678, -1.731827, -1.734925, -1.738201, -1.741003, -1.742933, -1.742847, -1.743328, -1.743713, -1.745154, -1.746409, -1.748076, -1.74978, -1.750643, -1.754186, -1.754986, -1.756397, -1.758024, -1.758979, -1.759065, -1.760624, -1.760972, -1.762637, -1.761787, -1.763726, -1.765543, -1.765016, -1.766732, -1.766754, -1.767378, -1.769156, -1.770782, -1.769529, -1.771681, -1.774107, -1.774083, -1.773465, -1.776551, -1.7769, -1.777184, -1.779577, -1.782635, -1.784107, -1.784463, -1.785458, -1.788683, -1.788266, -1.788353, -1.792286, -1.794119, -1.797406, -1.799931, -1.799882, -1.803332, -1.805629, -1.808943, -1.810944, -1.815338, -1.817579, -1.821914, -1.823939, -1.823984, -1.824479, -1.827874, -1.828624, -1.831189, -1.834249, -1.837352, -1.840545, -1.842513, -1.843883, -1.844658, -1.845469, -1.847506, -1.847783, -1.847724, -1.849609, -1.851567, -1.854874, -1.855014, -1.856372, -1.857242, -1.857328, -1.857547, -1.857453, -1.856168, -1.857152, -1.858451, -1.860661, -1.863533, -1.862458, -1.862873, -1.8625, -1.864446, -1.864005, -1.865644, -1.867303, -1.869859, -1.869177, -1.87106, -1.872557, -1.87485, -1.876792, -1.87792, -1.879416, -1.880891, -1.88229, -1.883001, -1.884895, -1.887511, -1.888618, -1.889667, -1.890988, -1.89195, -1.893431, -1.894883, -1.897578, -1.898132, -1.900848, -1.902939, -1.903204, -1.906468, -1.907731, -1.911094, -1.914545, -1.914069, -1.916715, -1.919814, -1.924357, -1.925624, -1.926027, -1.927533, -1.92878, -1.930781, -1.933259, -1.935024, -1.935669, -1.937159, -1.941593, -1.943703, -1.944188, -1.94607, -1.94767, -1.949901, -1.953692, -1.956016, -1.95587, -1.956956, -1.957812, -1.960381, -1.959847, -1.962302, -1.964968, -1.965408, -1.966073, -1.966652, -1.968157, -1.96777, -1.968737, -1.969974, -1.971081, -1.973194, -1.973107, -1.973395, -1.975831, -1.974888, -1.976667, -1.977967, -1.979229, -1.978025, -1.979688, -1.981466, -1.982145, -1.98411, -1.985344, -1.987456, -1.986855, -1.98958, -1.991533, -1.99268, -1.994391, -1.995883, -1.998483, -2.001424, -2.002542, -2.003317, -2.005271, -2.005408, -2.007813, -2.010125, -2.014482, -2.01531, -2.017421, -2.019714, -2.020994, -2.022138, -2.024231, -2.024747, -2.027357, -2.029235, -2.029265, -2.030994, -2.031304, -2.034138, -2.036861, -2.040324, -2.041713, -2.042037, -2.04359, -2.044022, -2.044908, -2.046657, -2.047824, -2.051014, -2.054657, -2.056817, -2.059453, -2.061589, -2.06364, -2.065237, -2.067247, -2.068725, -2.071458, -2.074905, -2.07737, -2.080565, -2.083697, -2.087481, -2.091082, -2.092851, -2.093103, -2.093195, -2.093516, -2.095365, -2.096425, -2.099223, -2.101484, -2.103373, -2.105643, -2.106495, -2.106768, -2.106139, -2.107027, -2.108662, -2.110675, -2.113137, -2.114984, -2.114976, -2.114794, -2.115665, -2.115897, -2.116617, -2.115794, -2.118241, -2.118774, -2.119518, -2.120522, -2.120542, -2.123268, -2.121393, -2.122028, -2.122763, -2.123667, -2.125674, -2.126533, -2.126987, -2.127242, -2.129283, -2.130683, -2.133371, -2.134053, -2.135321, -2.136652, -2.137676, -2.1401, -2.141002, -2.144012, -2.146379, -2.149109, -2.149892, -2.151595, -2.153952, -2.157497, -2.159382, -2.16167, -2.163208, -2.164861, -2.164779, -2.165491, -2.168431, -2.171925, -2.177754, -2.178715, -2.183376, -2.185389, -2.186762, -2.190714, -2.190458, -2.191987, -2.195885, -2.198871, -2.204202, -2.207521, -2.209987, -2.21454, -2.218014, -2.21995, -2.220463, -2.220907, -2.221254, -2.22355, -2.225333, -2.229345, -2.23353, -2.235106, -2.238055, -2.24006, -2.240727, -2.239621, -2.236791, -2.239479, -2.238161, -2.241344, -2.245895, -2.245886, -2.247513, -2.250166, -2.250099, -2.250016, -2.248876, -2.248007, -2.247105, -2.247338, -2.249197, -2.249319, -2.250475, -2.25188, -2.251492, -2.252683, -2.252503, -2.251842, -2.251578, -2.250173, -2.252358, -2.254551, -2.255458, -2.258278, -2.258637, -2.259614, -2.262342, -2.263566, -2.265738, -2.267658, -2.271066, -2.275012, -2.277248, -2.281006, -2.283612, -2.285054, -2.287975, -2.292252, -2.296906, -2.299709, -2.304351, -2.306453, -2.30684, -2.31102, -2.313174, -2.316671, -2.31785, -2.319218, -2.323156, -2.326314, -2.329258, -2.331731, -2.330921, -2.335348, -2.337216, -2.338341, -2.339784, -2.341652, -2.345573, -2.345867, -2.348178, -2.350725, -2.350301, -2.348484, -2.346947, -2.348321, -2.34914, -2.350959, -2.353362, -2.356062, -2.357188, -2.36042, -2.360488, -2.359332, -2.359335, -2.35875, -2.358047, -2.358225, -2.358656, -2.359831, -2.358635, -2.360408, -2.360445, -2.361667, -2.361858, -2.362926, -2.363986, -2.364288, -2.36439, -2.366317, -2.367123, -2.367277, -2.367964, -2.370787, -2.371625, -2.372217, -2.375174, -2.376335, -2.378235, -2.380094, -2.383183, -2.385061, -2.386831, -2.391057, -2.392312, -2.396703, -2.400629, -2.403565, -2.406785, -2.410075, -2.412154, -2.414591, -2.416001, -2.418411, -2.421814, -2.426937, -2.431327, -2.43597, -2.438255, -2.439214, -2.441636, -2.442908, -2.443591, -2.444271, -2.446042, -2.447553, -2.451574, -2.454322, -2.459259, -2.459167, -2.458988, -2.459791, -2.459803, -2.460155, -2.460693, -2.460836, -2.461752, -2.464313, -2.467197, -2.467691, -2.467576, -2.466714, -2.466182, -2.465541, -2.466343, -2.466851, -2.466728, -2.468352, -2.469074, -2.468673, -2.470402, -2.472062, -2.472489, -2.4717, -2.474044, -2.476117, -2.475176, -2.475954, -2.477194, -2.478101, -2.478769, -2.482395, -2.482993, -2.485696, -2.489882, -2.491889, -2.493382, -2.4963, -2.497217, -2.495696, -2.497921, -2.498425, -2.499485, -2.502473, -2.505013, -2.507983, -2.511344, -2.514346, -2.515093, -2.515869, -2.515267, -2.517344, -2.516297, -2.517832, -2.521177, -2.524304, -2.525843, -2.529733, -2.532366, -2.533173, -2.533271, -2.533655, -2.534038, -2.534921, -2.537768, -2.538384, -2.540839, -2.543183, -2.545565, -2.547411, -2.547801, -2.550262, -2.549876, -2.551255, -2.551288, -2.55151, -2.55373, -2.556228, -2.55787, -2.560246, -2.561557, -2.56405, -2.564885, -2.56686, -2.568948, -2.568611, -2.571201, -2.573409, -2.574788, -2.577568, -2.579327, -2.581748, -2.583365, -2.586189, -2.588238, -2.588712, -2.5902, -2.592187, -2.593757, -2.594959, -2.595729, -2.597616, -2.599509, -2.602154, -2.604658, -2.607614, -2.60966, -2.610898, -2.61283, -2.613601, -2.613473, -2.613544, -2.616515, -2.620266, -2.623817, -2.625905, -2.631148, -2.636015, 